vi "UHR-Fleezers Control (host) - 12.3.vi"() -> ()   [LabVIEW 2012] (continued)
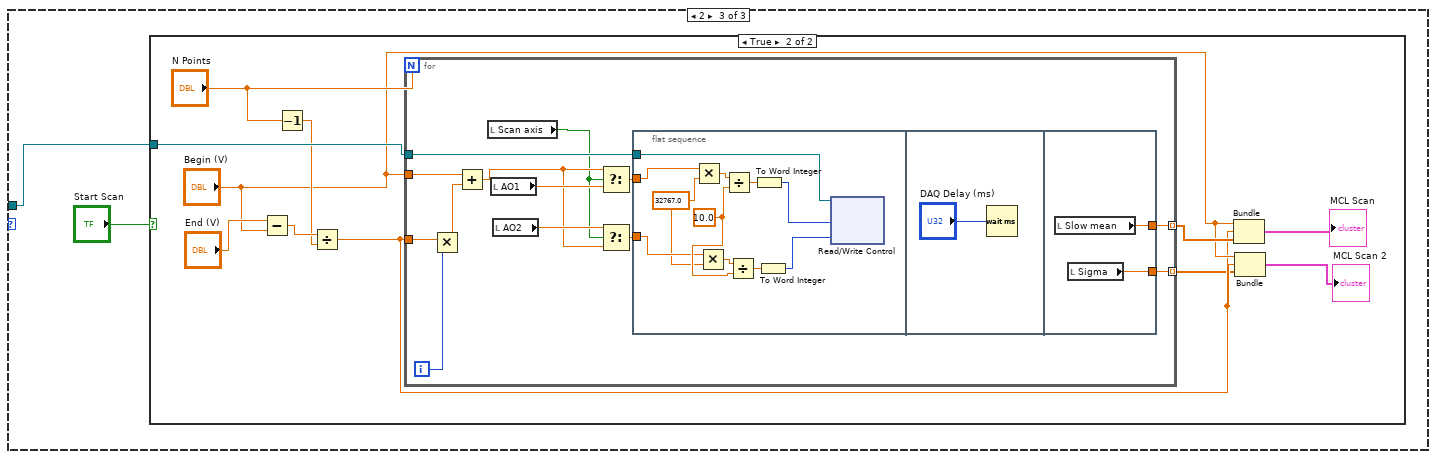
[diagram p3: hidden frame]
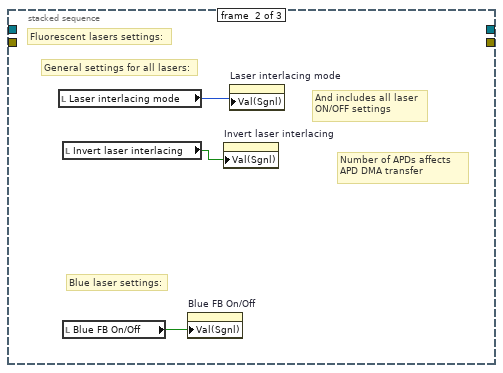
[diagram p5: hidden frame]
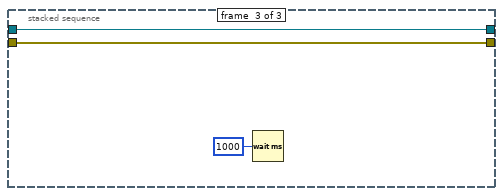
[diagram p6: hidden frame]
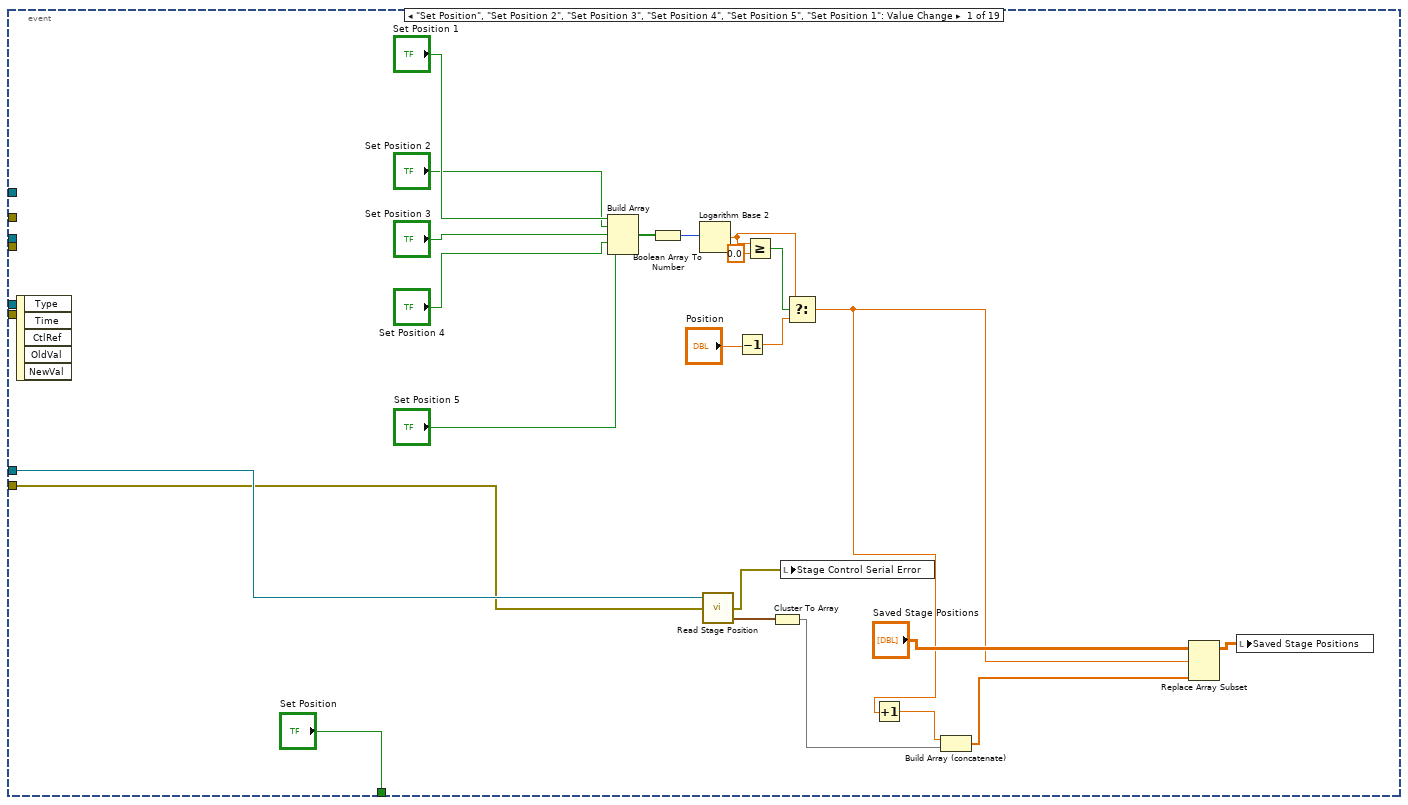
[diagram p8: hidden frame]
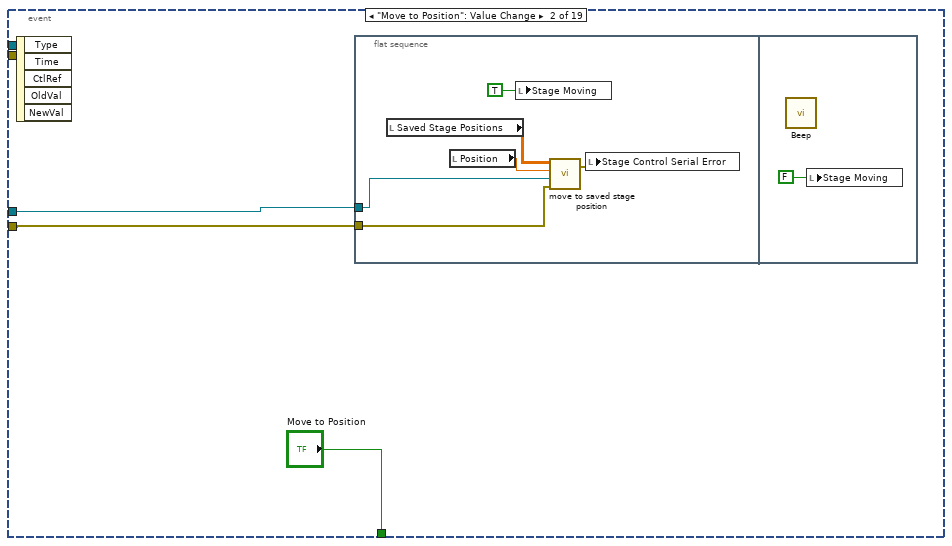
[diagram p9: hidden frame]
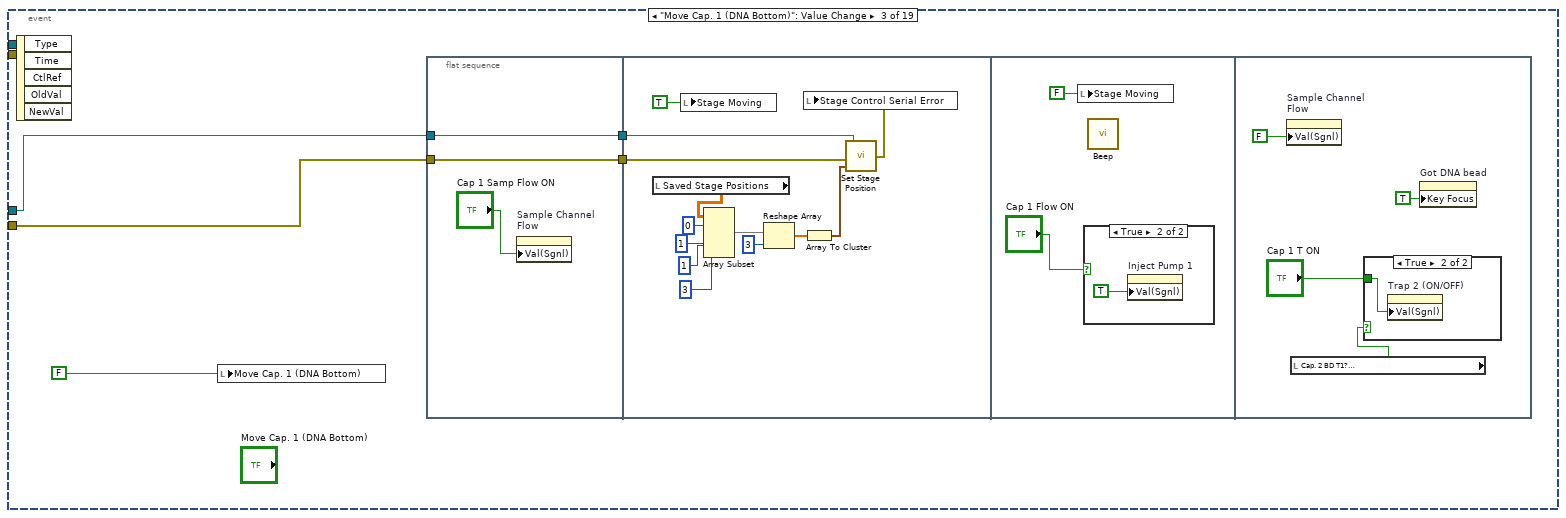
[diagram p10: hidden frame]
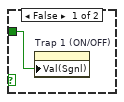
[diagram p12: hidden frame]
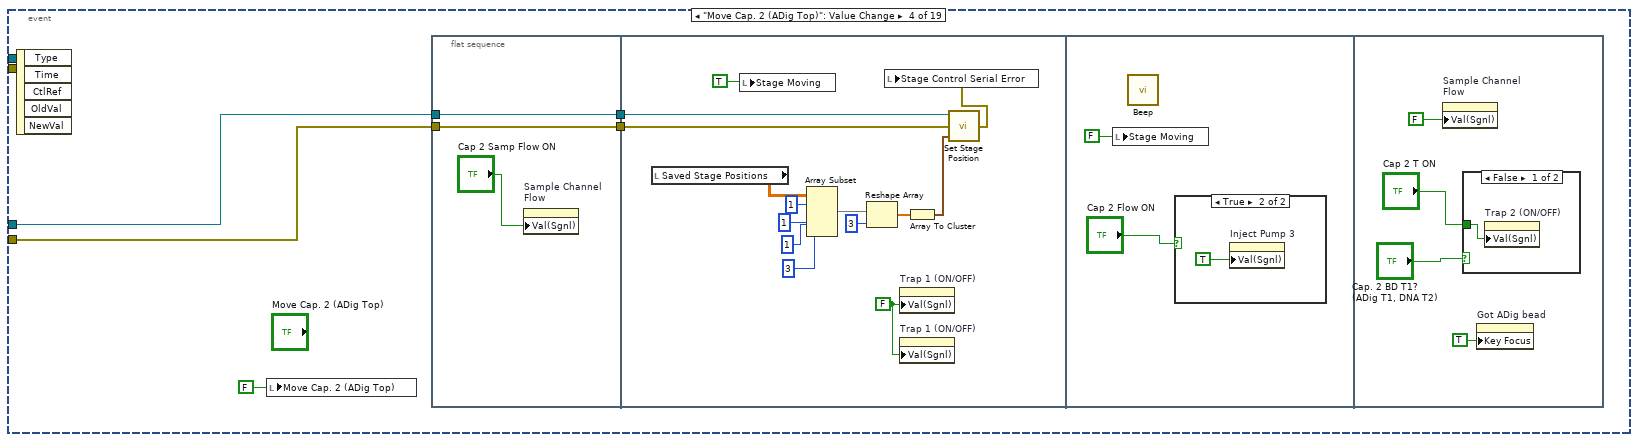
[diagram p13: hidden frame]
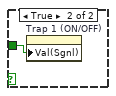
[diagram p15: hidden frame]
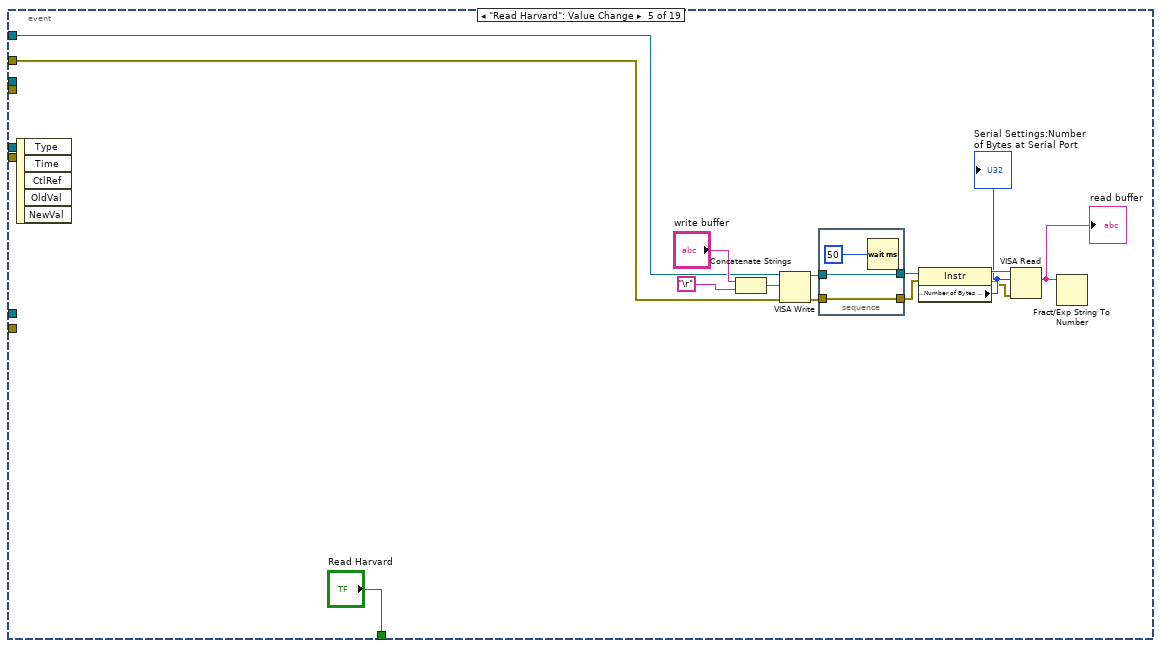
[diagram p16: hidden frame]
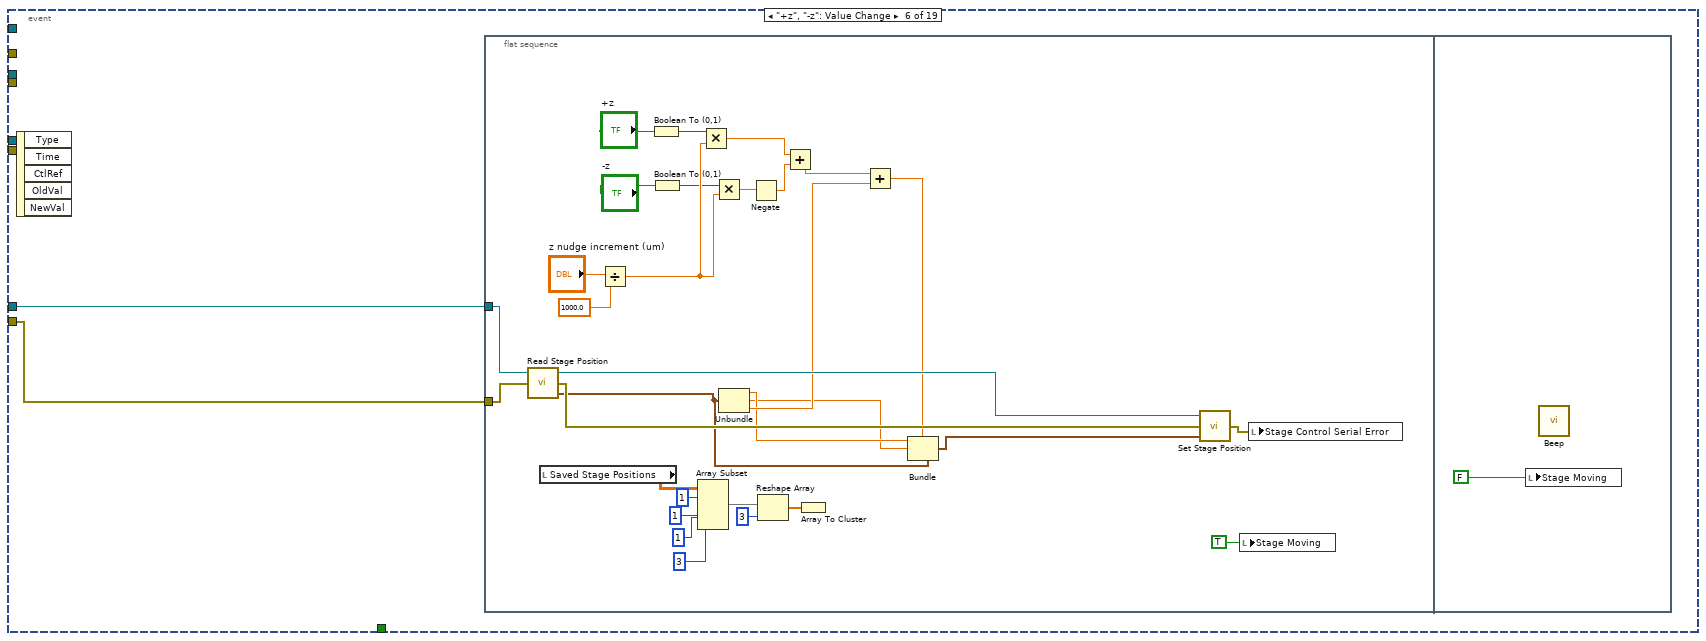
[diagram p17: hidden frame]
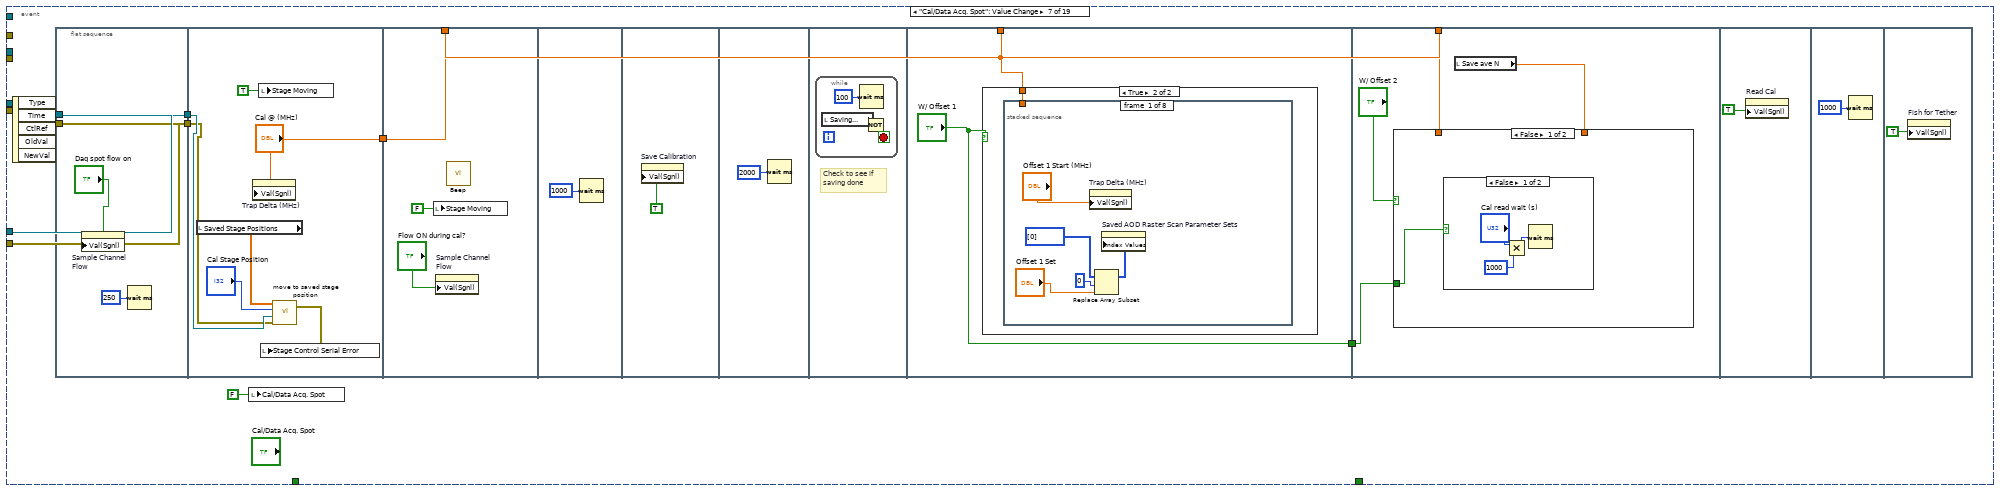
[diagram p18: hidden frame]
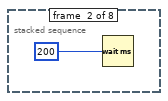
[diagram p20: hidden frame]
                n2922 = case "Write fl. data" shown="True" w4743 {
                  tunnel: w4742 -> [_ w4778]
                  tunnel: w4741 -> [_ w4777]
                  frame False {
                  }
                  frame True {
                    n2923 = Write to Binary File(file (use dialog)=w4778, data=w4777, 5:FALSE ("prepend array or string size? (T)"), 9:T25."big-endian, network order" ("byte order (0:big-endian, network order)")) -> ()  [unwired: 1 in, 4 out]
                  }
                }
                n2924 = Greater?(x="Save ave N", y=1.0) -> (0:w4747:bool)
                n2925 = Not(x=w4744) -> (.not. x?=w4746:bool)
                n2926 = And(x=w4746, y=w4747) -> (x .and. y?=w4694:bool)
                n2927 = case shown="True" w4694 {
                  tunnel: w4693 -> [w4758 w4769]
                  tunnel: [w4758 w4761] -> w4692
                  tunnel: "Save ave N" -> [_ w4762]
                  frame False {
                  }
                  frame True {
                    w4759 = 2 ("dimension size")
                    n2928 = Array Size(array=w4769) -> (size(s)=w4763:i32)
                    n2929 = Divide(x=w4763, y=w4759) -> (x/y=w4767:dbl)
                    n2930 = Reshape Array(w4769, w4767, w4759) -> (w4768:u64[][])
                    n2931 = Transpose 2D Array(2D array=w4768) -> (transposed array=w4766:u64[][])
                    n2932 = for {
                      tunnel: w4766 -> [w4771] mode=indexing
                      tunnel: [w4770] -> w4760 mode=indexing
                      tunnel: w4762 -> [w4772]
                      workers-P: _ -> [_]
                      n2933 = call "downsample 1D array - U64.vi"("Ave N"=w4772, "Array In"=w4771) -> ("Array Out"=w4770:u64[])  [unwired: 1 in]
                    }
                    n2934 = Transpose 2D Array(2D array=w4760) -> (transposed array=w4765:u64[][])
                    n2935 = Divide(x=w4763, y=w4762) -> (x/y=w4764:dbl)
                    n2936 = Reshape Array(w4765, w4764) -> (w4761:u64[])
                  }
                }
                n2937 = case shown="True" w4694 {
                  tunnel: w4749 -> [w4781 w4793]
                  tunnel: [w4781 w4785] -> w4745
                  tunnel: "Save ave N" -> [_ w4786]
                  tunnel: w4740 -> [_ w4784]
                  frame False {
                  }
                  frame True {
                    n2938 = Array Size(array=w4793) -> (size(s)=w4787:i32)
                    n2939 = Array Size(array=w4784) -> (size(s)=w4783:i32)
                    n2940 = Divide(x=w4787, y=w4783) -> (x/y=w4791:dbl)
                    n2941 = Reshape Array(w4793, w4791, w4783) -> (w4792:i16[][])
                    n2942 = Transpose 2D Array(2D array=w4792) -> (transposed array=w4790:i16[][])
                    n2943 = for {
                      tunnel: w4790 -> [w4796] mode=indexing
                      tunnel: [w4795] -> w4782 mode=indexing
                      tunnel: w4786 -> [w4794]
                      workers-P: _ -> [_]
                      n2944 = call "downsample 1D array - I16.vi"("Ave N"=w4794, "Array In"=w4796) -> ("Array Out"=w4795:i16[])  [unwired: 1 out]
                    }
                    n2945 = Transpose 2D Array(2D array=w4782) -> (transposed array=w4789:i16[][])
                    n2946 = Divide(x=w4787, y=w4786) -> (x/y=w4788:dbl)
                    n2947 = Reshape Array(w4789, w4788) -> (w4785:i16[])
                  }
                }
                n2948 = Index Array(array=w4680, index=2) -> (element=w4681:waveform(dbl))
                n2949 = Index Array(array=w4680, index=1) -> (element=w4714:waveform(dbl))
                n2950 = Index Array(array=w4680, index=0) -> (element=w4716:waveform(dbl))
                n2951 = Unbundle By Name(w4681) -> ("Y"=w4683:dbl[])
                n2952 = Unbundle By Name(w4714) -> ("Y"=w4718:dbl[])
                n2953 = Unbundle By Name(w4716) -> ("Y"=w4726:dbl[])
                n2954 = case "Write trap pos. data" shown="True" w4697 {
                  tunnel: w4696 -> [_ w4774]
                  tunnel: w4692 -> [_ w4773]
                  frame False {
                  }
                  frame True {
                    n2955 = Write to Binary File(file (use dialog)=w4774, data=w4773, 5:FALSE ("prepend array or string size? (T)"), 9:T25."big-endian, network order" ("byte order (0:big-endian, network order)")) -> ()  [unwired: 1 in, 4 out]
                  }
                }
                n2956 = Write to Binary File(file (use dialog)=w4752, data=w4745, 5:FALSE ("prepend array or string size? (T)"), 9:T25."big-endian, network order" ("byte order (0:big-endian, network order)")) -> ()  [unwired: 1 in, 4 out]
                n2957 = feedback #34(w4683) -> (w4684:dbl[])
                n2958 = Build Array (concatenate)(w4684, w4683) -> (w4679:dbl[])
                n2959 = Select(t=w4683, s=w4664, f=w4679) -> (s? t:f=w4669:dbl[])
                n2960 = feedback-in #34(w4669) -> ()
                n2961 = feedback #35(w4718) -> (w4720:dbl[])
                n2962 = Build Array (concatenate)(w4720, w4718) -> (w4719:dbl[])
                n2963 = Select(t=w4718, s=w4664, f=w4719) -> (s? t:f=w4708:dbl[])
                n2964 = feedback-in #35(w4708) -> ()
                n2965 = feedback #36(w4726) -> (w4739:dbl[])
                n2966 = Build Array (concatenate)(w4739, w4726) -> (w4738:dbl[])
                n2967 = Select(t=w4726, s=w4664, f=w4738) -> (s? t:f=w4713:dbl[])
                n2968 = feedback-in #36(w4713) -> ()
                n2969 = Divide(x=w4753, y=w4754) -> (x/y=w4756:dbl)
                n2970 = Multiply(x=w4756, y=100.0) -> (x*y=w4755:dbl)
                n2971 = Build Array(w4713, w4708, w4669) -> (→"Saved APD":dbl[][])
                n2972 = Array Size(array=w4713) -> (size(s)=w4731:i32)
                n2973 = Unbundle By Name(w4733) -> ("Y"=w4737:dbl[])
                n2974 = Subtract(x=w4731, y="N pts to average") -> (x-y=w4666:i32)
                n2975 = Multiply(x="N pts to average", y=u16 2) -> (x*y=w4709:u16)
                n2976 = Subtract(x=w4731, y=w4709) -> (x-y=w4667:i32)
                n2977 = feedback #37(w4737) -> (w4736:dbl[])
                n2978 = Build Array (concatenate)(w4736, w4737) -> (w4735:dbl[])
                n2979 = Select(t=w4737, s=w4664, f=w4735) -> (s? t:f=w4734:dbl[])
                "Trap Delta Graph" <- w4734
                n2980 = feedback-in #37(w4734) -> ()
                n2981 = Array Subset(array=w4713, index=w4666, length="N pts to average") -> (w4730:dbl[])
                n2982 = Array Subset(array=w4713, index=w4667, length="N pts to average") -> (w4729:dbl[])
                n2983 = Array Subset(array=w4708, index=w4666, length="N pts to average") -> (w4711:dbl[])
                n2984 = Array Subset(array=w4708, index=w4667, length="N pts to average") -> (w4710:dbl[])
                n2985 = Array Subset(array=w4669, index=w4666, length="N pts to average") -> (w4678:dbl[])
                n2986 = Array Subset(array=w4669, index=w4667, length="N pts to average") -> (w4677:dbl[])
                n2987 = Index Array(array=w4691, index=0) -> (element=w4689:waveform(dbl))
                n2988 = call-poly <vilib>:"Mean.vi"("X"=w4730) -> ("mean"=w4728:dbl)  [unwired: 1 out]
                n2989 = call-poly <vilib>:"Mean.vi"("X"=w4711) -> ("mean"=w4707:dbl)  [unwired: 1 out]
                n2990 = call-poly <vilib>:"Mean.vi"("X"=w4729) -> ("mean"=w4727:dbl)  [unwired: 1 out]
                n2991 = call-poly <vilib>:"Mean.vi"("X"=w4710) -> ("mean"=w4706:dbl)  [unwired: 1 out]
                n2992 = call-poly <vilib>:"Mean.vi"("X"=w4678) -> ("mean"=w4676:dbl)  [unwired: 1 out]
                n2993 = call-poly <vilib>:"Mean.vi"("X"=w4677) -> ("mean"=w4675:dbl)  [unwired: 1 out]
                n2994 = Unbundle By Name(w4689) -> ("Y"=w4687:dbl[])
                n2995 = Subtract(x=w4707, y=w4706) -> (x-y=w4698:dbl)
                "Delta Fl. 2" <- w4698
                n2996 = Subtract(x=w4676, y=w4675) -> (x-y=w4670:dbl)
                "Delta Fl. 3" <- w4670
                n2997 = Subtract(x=w4728, y=w4727) -> (x-y=w4725:dbl)
                "Delta Fl. 1" <- w4725
                n2998 = feedback #38(w4687) -> (w4686:dbl[])
                n2999 = Build Array (concatenate)(w4686, w4687) -> (w4688:dbl[])
                n3000 = Initialize Array(w4725, 1 ("dimension size")) -> (w4722:dbl[])
                n3001 = Initialize Array(w4698, 1 ("dimension size")) -> (w4703:dbl[])
                n3002 = Initialize Array(w4670, 1 ("dimension size")) -> (w4672:dbl[])
                n3003 = Select(t=w4687, s=w4664, f=w4688) -> (s? t:f=w4685:dbl[])
                "Saved trap pos" <- w4685
                n3004 = feedback-in #38(w4685) -> ()
                n3005 = feedback #39(w4722) -> (w4723:dbl[])
                n3006 = Build Array (concatenate)(w4723, w4722) -> (w4721:dbl[])
                n3007 = feedback #40(w4703) -> (w4704:dbl[])
                n3008 = feedback #41(w4672) -> (w4673:dbl[])
                n3009 = Build Array (concatenate)(w4704, w4703) -> (w4702:dbl[])
                n3010 = Build Array (concatenate)(w4673, w4672) -> (w4671:dbl[])
                n3011 = Select(t=w4722, s=w4664, f=w4721) -> (s? t:f=w4701:dbl[])
                n3012 = feedback-in #39(w4701) -> ()
                n3013 = Select(t=w4703, s=w4664, f=w4702) -> (s? t:f=w4700:dbl[])
                n3014 = feedback-in #40(w4700) -> ()
                n3015 = Select(t=w4672, s=w4664, f=w4671) -> (s? t:f=w4665:dbl[])
                n3016 = feedback-in #41(w4665) -> ()
                n3017 = Build Array(w4701, w4700, w4665) -> (→"Save APD Deriv":dbl[][])
              }
            }
            "Progress" <- w4647
            "Progress 2" <- w4647
          }
        }
      }
    }
    n3018 = local read "wait to reset values"() -> (w3308:bool)
    n3019 = Not(x=w3306) -> (.not. x?=w3309:bool)
    n3020 = And(x=w3309, y=w3308) -> (x .and. y?=w3310:bool)
    n3021 = case "Part of MCL raster scanning: returns to initial positions after scan done" shown="True" w3310 {
      tunnel: w3041 -> [w4186 w4193]
      tunnel: [w4186 w4192] -> w3312
      tunnel: w3040 -> [w4185 w4191]
      tunnel: [w4185 w4190] -> w3307
      frame False {
      }
      frame True {
        w4201 = 10.0 ("y")
        w4200 = 32767.0 ("y")
        # "to return scan values\nafter a synchronous \nAOM scan"
        n3022 = local read "AO2"() -> (w4194:dbl)
        n3023 = local read "AO1"() -> (w4195:dbl)
        n3024 = local write "wait to reset values"(FALSE ("wait to reset values")) -> ()
        n3025 = Multiply(x=w4195, y=w4200) -> (x*y=w4197:dbl)
        n3026 = Multiply(x=w4194, y=w4200) -> (x*y=w4199:dbl)
        n3027 = Divide(x=w4197, y=w4201) -> (x/y=w4196:dbl)
        n3028 = Divide(x=w4199, y=w4201) -> (x/y=w4198:dbl)
        n3029 = To Word Integer(number=w4196) -> (16bit integer=w4202:i16)
        n3030 = To Word Integer(number=w4198) -> (16bit integer=w4203:i16)
        n3031 = local read "Total Counts (ticks)"() -> (w4187:u16)
        n3032 = xnode "Read/Write Control"("FPGA VI Reference In"=w4193, "error in"=w4191, "AO1"=w4202, "AO2"=w4203, "MCL count"=w4187) -> ("FPGA VI Reference Out"=w4192:T19, "error out"=w4190:errorcluster)
        n3033 = local read "Scan Range (V)\n(of steps)"() -> (w4188:dbl)
        n3034 = property on="Scan Range (V)\n(of steps)" class="DigNum (strict)"("Val(Sgnl)"=w4188) -> ()  [unwired: 2 in, 2 out]
      }
    }
    n3035 = node-c288() -> ()  [unwired: 2 out]
  }
  n3036 = flat-sequence "Video" {
    tunnel: [w4806] -> w110
    tunnel: w110 -> [w4846]
    frame #0 {
      n3037 = while {
        stop <- w4798 continue-if-true
        n3038 = call "Close Video Capture.vi"() -> ("error code OUT"=w4800:i32)
        n3039 = Equal?(x=w4800, y=0) -> (x = y?=w4798:bool)
      }
      n3040 = local write "Stop All"(FALSE ("Stop All")) -> ()
    }
    frame #1 {
      n3041 = call "DMR_Init.vi"() -> ()  [unwired: 3 out]
    }
    frame #2 {
      w4801 = "DE245428202"  # MSU fleezers card #
      (unwired) "DE019116701"  # Illinois fleezers card #
      # "Setting the destination format to Mono8 makes sure that the image can be displayed in the intensity plot."
      n3042 = call "DMR_GetDevice.vi"("search string IN"=w4801) -> ("device handle OUT"=w4824:i32)  [unwired: 4 in, 2 out]
      n3043 = call "DMR_OpenDevice.vi"("device handle IN"=w4824) -> ("driver handle OUT"=w4807:i32)  [unwired: 4 out]
      n3044 = call "DMR_FindList.vi"("flags IN"=u32 0 ("flags"), "list name IN"="" ("String"), "list type IN"=T44."camera descriptions", "driver handle IN"=w4807) -> ("list handle OUT"=w4810:i32)  [unwired: 2 out]
      n3045 = call "DMR_FindList.vi"("flags IN"=u32 0 ("flags"), "list name IN"="Base", "list type IN"=T44."setting", "driver handle IN"=w4807) -> ("list handle OUT"=w4808:i32)  [unwired: 2 out]
      n3046 = call "OBJ_GetHandle.vi"("object name IN"="VideoStandard", "list handle IN"=w4810) -> ("object handle OUT"=w4804:i32)  [unwired: 3 out]
      n3047 = call "OBJ_GetHandle.vi"("object name IN"="PixelFormat", "list handle IN"=w4808) -> ("object handle OUT"=w4818:i32)  [unwired: 3 out]
      n3048 = call "OBJ_SetS.vi"("value index IN"=0, "value IN"="NTSC M", "object handle IN"=w4804) -> ()  [unwired: 2 out]
      n3049 = call "OBJ_SetS.vi"("value index IN"=0, "value IN"="Mono8" ("value"), "object handle IN"=w4818) -> ()  [unwired: 2 out]
      n3050 = call "OBJ_GetHandle.vi"("object name IN"="VideoChannel", "list handle IN"=w4808) -> ("object handle OUT"=w4814:i32)  [unwired: 3 out]
      n3051 = while {
        tunnel: [w4828] -> w4806
        tunnel: w4807 -> [w4825]
        stop <- w4826 continue-if-true
        n3052 = call "DMR_ImageRequestSingle.vi"("request control IN"=0, "driver handle IN"=w4825) -> ("error code OUT"=w4827:i32, "driver handle OUT"=w4828:i32)  [unwired: 2 out]
        n3053 = Equal To 0?(x=w4827) -> (x = 0?=w4826:bool)
      }
      n3054 = call "OBJ_SetI.vi"("value index IN"=0, "value IN"=3 ("Video channel"), "object handle IN"=w4814) -> ()  [unwired: 2 out]
    }
    frame #3 {
      w4834 = T17 0 items=["Grayscale (U8)", "Grayscale (I16)", "Grayscale (SGL)", "Complex (CSG)", "RGB (U32)", "HSL (U32)", "RGB (U64)"] ("Image Type")
      w4842 = T17 0 items=["Grayscale (U8)", "Grayscale (I16)", "Grayscale (SGL)", "Complex (CSG)", "RGB (U32)", "HSL (U32)", "RGB (U64)"] ("Image Type")
      n3055 = for "Create Greyscale map" {
        N: 256 -> [_]
        tunnel: [w4848] -> w4831 mode=indexing
        workers-P: _ -> [_]
        i -> [w4851]
        n3056 = To Unsigned Byte Integer(number=w4851) -> (unsigned 8bit integer=w4847:u8)
        n3057 = Join Numbers(hi=w4847, lo=w4847) -> ((hi.lo)=w4850:u16)
        n3058 = Join Numbers(hi=w4847, lo=w4847) -> ((hi.lo)=w4849:u16)
        n3059 = Join Numbers(hi=w4850, lo=w4849) -> ((hi.lo)=w4848:u32)
      }
      n3060 = call "IMAQ Create"("Image Name"="Scaled video", "Image Type"=w4834) -> ("New Image"=w4833:T2)  [unwired: 2 in, 2 out]
      n3061 = call "IMAQ Create"("Image Name"="Main video", "Image Type"=w4842) -> ("New Image"=w4843:T2)  [unwired: 2 in, 2 out]
      n3062 = node-c288(0 ("Processor")) -> (w4841:T21)  [unwired: 3 out]
      n3063 = Initialize Array(u32 0 ("Window Number (0...15)"), 480 ("dimension size"), 640 ("dimension size")) -> (w4836:u32[][])
      n3064 = timed-loop {
        tunnel: w4846 -> [w4868]
        tunnel: [w4867] -> w4845
        tunnel: w4843 -> [w4866]
        timing: w4841 -> [_]
        timing-out: [_] -> w4840
        tunnel: w4836 -> [w4855]
        tunnel: w4833 -> [w4853]
        tunnel: w4831 -> [w4852]
        stop <- w4854 stop-if-true
        # "This block performs the \nactual image capture."
        n3065 = node-c288() -> ()  [unwired: 2 out]
        n3066 = local read "Stop All"() -> (w4854:bool)
        n3067 = Reciprocal(x="Video Capture Rate (Hz)") -> (1/x=w4858:dbl)
        n3068 = Multiply(x=w4858, y=1000.0) -> (x*y=w4856:dbl)
        n3069 = call "DMR_ImageRequestWaitFor.vi"("queue number IN"=0, "timeout(ms) IN"=500, "driver handle IN"=w4868) -> ("error code OUT"=w4872:i32, "request number OUT"=w4869:i32, "driver handle OUT"=w4870:i32)
        n3070 = feedback #42(T45 refnum ("Avi Refnum")) -> (w4860:T45)
        n3071 = case shown="True" "New Video File" {
          tunnel: [T45 refnum ("Avi Refnum") w4889] -> w4862
          tunnel: [FALSE TRUE] -> w4863
          tunnel: w4860 -> [_ w4885]
          frame False {
          }
          frame True {
            n3072 = call "Create new save file.vi"("Ext"=".avi" ("string"), "Index In"="Video Index") -> ("Path Out"=w4881:path, "Index Out"=w4882:dbl)  [unwired: 1 in]
            "Path Out" <- w4881
            n3073 = Not Equal?(x=w4885, y=T45 refnum ("Avi Refnum")) -> (x != y?=w4886:bool)
            n3074 = Increment(x=w4882) -> (x+1=w4891:dbl)
            n3075 = case shown="True" w4886 {
              tunnel: w4885 -> [_ w4892]
              frame False {
              }
              frame True {
                n3076 = call "IMAQ AVI Close"("Avi Refnum"=w4892) -> ()  [unwired: 1 in, 10 out]
              }
            }
            n3077 = local write "Video Index"(w4891) -> ()
            n3078 = call "IMAQ AVI Create"("Frames Per Second"=u32 30, "AVI Path"=w4881) -> ("Avi Refnum"=w4889:T45)  [unwired: 5 in, 4 out]
          }
        }
        n3079 = Equal To 0?(x=w4872) -> (x = 0?=w4871:bool)
        n3080 = Select(t=w4862, s=w4863, f=w4860) -> (s? t:f=w4861:T45)
        n3081 = feedback-in #42(w4861) -> ()
        n3082 = case shown="True" w4871 {
          tunnel: w4870 -> [w4893 w4938]
          tunnel: w4869 -> [_ w4937]
          tunnel: [w4893 w4934] -> w4867
          tunnel: w4866 -> [_ w4919]
          tunnel: w4855 -> [_ w4923]
          tunnel: w4861 -> [_ w4921]
          tunnel: w4853 -> [_ w4916]
          tunnel: w4852 -> [_ w4915]
          frame False {
          }
          frame True {
            w4928 = u32 0 ("X-offset IN")
            n3083 = call "DMR_GetImageRequestBufferData.vi"("driver handle IN"=w4938, "request number IN"=w4937) -> ("width OUT"=w4927:i32, "height OUT"=w4926:i32, "driver handle OUT"=w4933:i32, "request number OUT"=w4932:i32, "bytes per pixel OUT"=w4929:i32)  [unwired: 13 out]
            n3084 = call "DMR_GetImageRequestBufferImageData.vi"("driver handle IN"=w4933, "request number IN"=w4932, "bytes per pixel IN"=w4929, "X-offset IN"=w4928, "Y-offset IN"=w4928, "height IN"=w4926, "width IN"=w4927) -> ("driver handle OUT"=w4931:u32, "request number OUT"=w4930:u32, "image OUT"=w4896:u32[][])  [unwired: 10 out]
            n3085 = Transpose 2D Array(2D array=w4896) -> (transposed array=w4902:u32[][])
            n3086 = Select(t=w4902, s="Flip Y (or X)", f=w4896) -> (s? t:f=w4901:u32[][])
            n3087 = call "DMR_ImageRequestUnlock.vi"("request number IN"=w4930, "driver handle IN"=w4931) -> ("driver handle OUT"=w4936:i32)  [unwired: 1 in, 2 out]
            n3088 = for {
              tunnel: w4901 -> [w4940] mode=indexing
              tunnel: [w4939] -> w4899 mode=indexing
              n3089 = Reverse 1D Array(array=w4940) -> (reversed array=w4939:u32[])
            }
            n3090 = call "DMR_ImageRequestSingle.vi"("request control IN"=0, "driver handle IN"=w4936) -> ("driver handle OUT"=w4934:i32)  [unwired: 3 out]
            n3091 = Transpose 2D Array(2D array=w4899) -> (transposed array=w4900:u32[][])
            n3092 = Select(t=w4900, s="Flip Y (or X)", f=w4899) -> (s? t:f=w4897:u32[][])
            n3093 = Select(t=w4897, s="Flip Image", f=w4896) -> (s? t:f=w4894:u32[][])
            n3094 = case shown="True" "Averaging" {
              tunnel: w4894 -> [w4962 w4967]
              tunnel: [w4962 w4966] -> w4920
              tunnel: w4923 -> [_ w4964]
              frame False {
              }
              frame True {
                (unwired) 1
                w4972 = 1
                n3095 = feedback #43(w4964) -> (w4963:u32[][])
                n3096 = Add(x=w4967, y=w4963) -> (x+y=w4968:u32[][])
                n3097 = Select(t=w4964, s="Reset Averaging", f=w4968) -> (s? t:f=w4970:u32[][])
                n3098 = feedback-in #43(w4970) -> ()
                n3099 = feedback #44(w4972) -> (w4965:i32)
                n3100 = Divide(x=w4968, y=w4965) -> (x/y=w4969:dbl[][])
                n3101 = Increment(x=w4965) -> (x+1=w4973:i32)
                n3102 = To Unsigned Long Integer(number=w4969) -> (unsigned 32bit integer=w4966:u32[][])
                n3103 = Select(t=w4972, s="Reset Averaging", f=w4973) -> (s? t:f=w4971:i32)
                n3104 = feedback-in #44(w4971) -> ()
              }
            }
            n3105 = To Double Precision Float(number=w4920) -> (double precision float=w4913:dbl[][])
            n3106 = In Range and Coerce(upper limit="Intensity Upper", x=w4913, lower limit="Intensity Lower") -> (coerced(x)=w4912:dbl[][])  [unwired: 1 out]
            n3107 = Subtract(x="Intensity Upper", y="Intensity Lower") -> (x-y=w4909:dbl)
            n3108 = Subtract(x=w4912, y="Intensity Lower") -> (x-y=w4910:dbl[][])
            n3109 = Divide(x=w4910, y=w4909) -> (x/y=w4911:dbl[][])
            n3110 = To Unsigned Byte Integer(number=w4920) -> (unsigned 8bit integer=w4918:u8[][])
            n3111 = Multiply(x=255.0, y=w4911) -> (x*y=w4907:dbl[][])
            n3112 = call "IMAQ ArrayToImage"("Image Pixels (U8)"=w4918, "Image"=w4919) -> ("Image Out"=w4917:T2)  [unwired: 4 in, 5 out]
            "Primary Video Display" <- w4917
            n3113 = To Unsigned Byte Integer(number=w4907) -> (unsigned 8bit integer=w4914:u8[][])
            n3114 = call "IMAQ ArrayToImage"("Image Pixels (U8)"=w4914, "Image"=w4916) -> ("Image Out"=w4903:T2)  [unwired: 4 in, 5 out]
            n3115 = First Call?() -> (First Call?: T/F=w4904:bool)
            n3116 = case shown="True" "Save Video" {
              tunnel: w4921 -> [_ w4961]
              tunnel: w4917 -> [_ w4960]
              frame False {
              }
              frame True {
                n3117 = call "IMAQ AVI Write Frame"("Image"=w4960, "Avi Refnum"=w4961) -> ()  [unwired: 2 in, 8 out]
              }
            }
            n3118 = case shown="True" w4904 {
              tunnel: w4903 -> [w4941 w4952]
              frame False {
                n3119 = flat-sequence {
                  tunnel: w4941 -> [w4947]
                  frame #0 {
                    w4944 = FALSE ("Get/Set Status? (Set)")
                    w4943 = 0 ("Window Number (0...15)")
                    n3120 = call "IMAQ WindSize"("Get/Set Status? (Set)"=w4944, "Window Number"=w4943) -> ("Width & Height out"=→"Window Size":cluster{"Width":i32, "Height":i32})  [unwired: 4 in, 2 out]
                    n3121 = call "IMAQ WindMove"("Window Number (0...15)"=w4943, "Get/Set Status? (Set)"=w4944) -> ("Coordinates (screen)"=→"Window Position":cluster{"X Position":i32, "Y Position":i32})  [unwired: 3 in, 1 out]
                    n3122 = call "IMAQ WindDraw"("Resize to Image Size? (Y)"=FALSE, "Window Number (0...15)"=w4943, "Image"=w4947) -> ()  [unwired: 7 in, 2 out]
                  }
                  frame #1 {
                    n3123 = call "IMAQ WindZoom 2"("Center Point"="Center Point", "Zoom to Fit? (False)"=FALSE, "Zoom Factor"="Zoom Factor") -> ()  [unwired: 5 in, 4 out]
                  }
                }
              }
              frame True {
                n3124 = flat-sequence {
                  tunnel: w4952 -> [w4955]
                  tunnel: [w4953] -> w4951
                  tunnel: w4951 -> [w4957]
                  frame #0 {
                    w4954 = TRUE ("Resize to Image Size? (Y)")
                    w4953 = 0 ("Window Number (0...15)")
                    n3125 = call "IMAQ WindNonTearing"("Window Number"=w4953, "NonTearing? (True)"=w4954) -> ()  [unwired: 8 in, 2 out]
                    n3126 = call "IMAQ WindDraw"("Resize to Image Size? (Y)"=w4954, "Window Number (0...15)"=w4953, "Image"=w4955) -> ()  [unwired: 7 in, 2 out]
                  }
                  frame #1 {
                    n3127 = call "IMAQ WindSize"("Scrollbars? (N)"=FALSE, "Width & Height"="Initial Window Size", "Window Number"=w4957) -> ()  [unwired: 3 in, 3 out]
                    n3128 = call "IMAQ WindMove"("Window Number (0...15)"=w4957, "Coordinates (screen)"="Initial Window Position") -> ()  [unwired: 3 in, 2 out]
                  }
                }
              }
            }
            n3129 = case shown="True" "Save Image" {
              tunnel: w4918 -> [_ w4976]
              tunnel: w4915 -> [_ w4975]
              frame False {
              }
              frame True {
                n3130 = call <vilib>:"Flatten Pixmap.vi"("colors"=w4975, "8-bit pixmap"=w4976) -> ("image data"=w4982:T46)  [unwired: 4 in, 5 out]
                n3131 = call "Create new save file.vi"("Insert"="video_frame_" ("string"), "Ext"=".bmp" ("string"), "Index In"="Image Index") -> ("Path Out"=w4978:path, "Index Out"=w4983:dbl)
                n3132 = Increment(x=w4983) -> (x+1=w4977:dbl)
                n3133 = local write "Image Index"(w4977) -> ()
                n3134 = call <vilib>:"Write BMP File.vi"("image data"=w4982, "path to BMP file"=w4978) -> ()  [unwired: 1 in, 9 out]
              }
            }
          }
        }
        n3135 = node-c288(w4856) -> ()  [unwired: 1 out]
      }
      n3136 = node-c288(w4840) -> ()  [unwired: 1 out]
      n3137 = call "DMR_CloseDevice.vi"("driver handle IN"=w4845) -> ()  [unwired: 1 in, 4 out]
    }
    frame #4 {
      n3138 = call "DMR_Close.vi"() -> ()  [unwired: 1 out]
    }
  }
  n3139 = timed-loop "Rough control of MCL mirror stage (debugging)" {
    tunnel: w8 -> [w4990]
    tunnel: [w4989] -> w250
    timing: w2 -> [_]
    timing-out: [_] -> w1
    stop <- w4989 stop-if-true
    n3140 = node-c288() -> ()  [unwired: 2 out]
    n3141 = case shown="1" "MCL Mode" {
      tunnel: w4990 -> [_ w4993 w5040]
      frame 0, Default {
      }
      frame 1 {
        n3142 = node-c288() -> (w4995:T21)  [unwired: 4 out]
        n3143 = timed-loop "Oscillate MCL mirror" {
          timing: w4995 -> [_]
          timing-out: [_] -> w4994
          tunnel: w4993 -> [w5034]
          i -> [w5033]
          stop <- w4996 stop-if-true
          n3144 = node-c288() -> (w5032:i64)  [unwired: 1 out]
          n3145 = Multiply(x="AO1", y=32767.0) -> (x*y=w5028:dbl)
          n3146 = Multiply(x="AO2", y=32767.0) -> (x*y=w5023:dbl)
          n3147 = Divide(x=w5028, y=10.0) -> (x/y=w5029:dbl)
          n3148 = Divide(x=w5023, y=10.0) -> (x/y=w5024:dbl)
          n3149 = To Word Integer(number=w5029) -> (16bit integer=w5021:i16)
          n3150 = To Word Integer(number=w5024) -> (16bit integer=w5020:i16)
          n3151 = Divide(x=w5032, y=i64 1000) -> (x/y=w5003:dbl)
          n3152 = Multiply(x=w5003, y=w5033) -> (x*y=w5014:dbl)
          n3153 = Multiply(x="Osc. freq. (Hz) 2", y=6.283185307179586) -> (x*y=w5015:dbl)
          n3154 = Multiply(x=w5015, y=w5014) -> (x*y=w5013:dbl)
          n3155 = Sine(x=w5013) -> (sin(x)=w5012:dbl)
          n3156 = Multiply(x=w5012, y="Osc. amp. (V)") -> (x*y=w5010:dbl)
          n3157 = Add(x=w5010, y="Osc. center (V)") -> (x+y=w5008:dbl)
          n3158 = Divide(x=w5008, y=10.0) -> (x/y=w5006:dbl)
          n3159 = Multiply(x=w5006, y=32767.0) -> (x*y=w5001:dbl)
          n3160 = Select(t=w5001, s="Scan axis", f=w5021) -> (s? t:f=w5019:dbl)
          n3161 = Select(t=w5020, s="Scan axis", f=w5001) -> (s? t:f=w5018:dbl)
          n3162 = local read "MCL Mode"() -> (w5000:u16)
          n3163 = Not Equal?(x=w5000, y=u16 1) -> (x != y?=w4997:bool)
          n3164 = local read "Stop All"() -> (w4998:bool)
          n3165 = xnode "Read/Write Control"("FPGA VI Reference In"=w5034, "AO1"=w5019, "AO2"=w5018) -> ()  [unwired: 1 in, 2 out]
          n3166 = Compound Arithmetic op=OR(w4998, w4997) -> (w4996:bool)
          n3167 = node-c288() -> ()  [unwired: 2 out]
        }
        n3168 = node-c288(w4994) -> ()  [unwired: 1 out]
      }
      frame 2 {
        n3169 = case shown="True" "Start Scan" {
          tunnel: w5040 -> [_ w5052]
          frame False {
          }
          frame True {
            n3170 = Subtract(x="End (V)", y="Begin (V)") -> (x-y=w5048:dbl)
            n3171 = Decrement(x="N Points") -> (x-1=w5047:dbl)
            n3172 = Divide(x=w5048, y=w5047) -> (x/y=w5045:dbl)
            n3173 = for {
              N: "N Points" -> [_]
              tunnel: "Begin (V)" -> [w5065]
              tunnel: w5052 -> [w5057]
              tunnel: [w5056] -> w5051 mode=indexing
              tunnel: w5045 -> [w5055]
              tunnel: [w5053] -> w5044 mode=indexing
              i -> [w5064]
              n3174 = Multiply(x=w5055, y=w5064) -> (x*y=w5063:dbl)
              n3175 = Add(x=w5065, y=w5063) -> (x+y=w5060:dbl)
              n3176 = local read "Scan axis"() -> (w5054:bool)
              n3177 = local read "AO1"() -> (w5062:dbl)
              n3178 = local read "AO2"() -> (w5061:dbl)
              n3179 = Select(t=w5060, s=w5054, f=w5062) -> (s? t:f=w5059:dbl)
              n3180 = Select(t=w5061, s=w5054, f=w5060) -> (s? t:f=w5058:dbl)
              n3181 = flat-sequence {
                tunnel: w5059 -> [w5069]
                tunnel: w5058 -> [w5068]
                tunnel: w5057 -> [w5066]
                tunnel: [w5079] -> w5056
                tunnel: [w5078] -> w5053
                frame #0 {
                  w5072 = 10.0 ("y")
                  w5067 = 32767.0 ("y")
                  n3182 = Multiply(x=w5069, y=w5067) -> (x*y=w5075:dbl)
                  n3183 = Multiply(x=w5068, y=w5067) -> (x*y=w5073:dbl)
                  n3184 = Divide(x=w5075, y=w5072) -> (x/y=w5076:dbl)
                  n3185 = Divide(x=w5073, y=w5072) -> (x/y=w5074:dbl)
                  n3186 = To Word Integer(number=w5076) -> (16bit integer=w5070:i16)
                  n3187 = To Word Integer(number=w5074) -> (16bit integer=w5071:i16)
                  n3188 = xnode "Read/Write Control"("FPGA VI Reference In"=w5066, "AO1"=w5070, "AO2"=w5071) -> ()  [unwired: 1 in, 2 out]
                }
                frame #1 {
                  n3189 = Wait (ms)(milliseconds to wait="DAQ Delay (ms)") -> ()  [unwired: 1 out]
                }
                frame #2 {
                  n3190 = local read "Slow mean"() -> (w5079:dbl)
                  n3191 = local read "Sigma"() -> (w5078:dbl)
                }
              }
            }
            n3192 = Bundle("Begin (V)"="Begin (V)", w5045, w5051) -> (→"MCL Scan":cluster{"Begin (V)":dbl, dbl, dbl[]})  [unwired: 1 out]
            n3193 = Bundle("Begin (V)"="Begin (V)", w5045, w5044) -> (→"MCL Scan 2":cluster{"Begin (V)":dbl, dbl, dbl[]})  [unwired: 1 out]
          }
        }
      }
    }
    n3194 = local read "Stop All"() -> (w4989:bool)
    n3195 = node-c288() -> ()  [unwired: 2 out]
  }
  n3196 = node-c288(w1) -> ()  [unwired: 1 out]
  n3197 = node-c288(w121) -> ()  [unwired: 1 out]
  n3198 = node-c288(w123) -> ()  [unwired: 1 out]
  n3199 = property on="Saved trap pos" class="WFGraph (strict)"("Visible"=FALSE) -> ()  [unwired: 2 in, 2 out]
  n3200 = property on="Trap Delta Graph" class="WFGraph (strict)"("Visible"=TRUE) -> ()  [unwired: 2 in, 2 out]
  n3201 = node-c288(w108) -> ()  [unwired: 1 out]
  n3202 = local write "Trap pos"(FALSE ("Trap pos")) -> ()
  n3203 = disable-structure shown="Disabled" {
    disable-tunnel: w112 -> [w5081 _]
    disable-tunnel: w111 -> [w5080 _]
    frame Disabled {
      n3204 = VISA Close(VISA resource name=w5081, error in (no error)=w5080) -> (error out=w5082:errorcluster)
      n3205 = call <vilib>:"Simple Error Handler.vi"("error in (no error)"=w5082) -> ()  [unwired: 1 in, 8 out]
    }
    frame Enabled {
    }
  }
  n3206 = node-c288(w194) -> ()  [unwired: 1 out]
  n3207 = node-c288(w119) -> ()  [unwired: 1 out]
  n3208 = flat-sequence {
    tunnel: w285 -> [w5086]
    tunnel: w287 -> [w5087]
    tunnel: [w5085] -> w266
    tunnel: [w5084] -> w265
    tunnel: w250 -> [_]
    tunnel: w202 -> [_]
    tunnel: w125 -> [_]
    tunnel: w266 -> [w5088]
    tunnel: w265 -> [w5089]
    frame #0 {
      w5083 = FALSE ("AI to FIFO")
      n3209 = xnode "Read/Write Control"("FPGA VI Reference In"=w5087, "error in"=w5086, "AI to FIFO"=w5083, "APD to FIFO"=w5083) -> ("FPGA VI Reference Out"=w5085:T19, "error out"=w5084:errorcluster)
    }
    frame #1 {
      n3210 = xnode "Close FPGA VI Reference"("FPGA VI Reference In"=w5088, "error in"=w5089) -> ("error out"=→"error out":errorcluster)
    }
  }
